vi "Dresden R2R Sputter 03.02.2018 IY24.vi"() -> ()   [LabVIEW 2009] (continued)
                                n18827 = local write "Error Message"("Shut Down Process  cancelled\nbecause  CH-VBV  not opened.\nPlease check CH-VBV2 connections." ("Error Message")) -> ()
                                n18828 = local write "Semi"(TRUE ("Semi")) -> ()
                                }
                                }
                                n18829 = local read "Ch2_Ch_vbv_di"() -> (w25328:bool)
                                n18830 = case shown="False" w25328 {
                                tunnel: [FALSE TRUE] -> w25330
                                frame #0 {
                                n18831 = local write "Ch2_Ch_vbv_do"(TRUE ("Ch1_Ch_cc_on_off_di")) -> ()
                                n18832 = Wait Until Next ms Multiple(millisecond multiple=u32 500) -> ()  [unwired: 1 out]
                                }
                                frame #1 {
                                }
                                }
                                n18833 = local read "Semi"() -> (w25331:bool)
                                n18834 = Or(x=w25330, y=w25331) -> (x .or. y?=w25329:bool)
                                }
                                }
                                frame #1 {
                                }
                                }
                                }
                                frame #1 {
                                n18835 = local read "Semi"() -> (w25341:bool)
                                n18836 = case shown="False" w25341 {
                                frame #0 {
                                n18837 = local write "Ch2_Sd13"(TRUE ("Ch1_Sd12")) -> ()
                                n18838 = Wait (ms)(milliseconds to wait=u32 1000) -> ()  [unwired: 1 out]
                                }
                                frame #1 {
                                }
                                }
                                }
                                }
                                }
                                frame #1 {
                                }
                                }
                                }
                                }
                              }
                              frame #13 {
                                # "TRNS GV-BP2 OPEN"
                                n18839 = local read "Yes 2"() -> (w25344:bool)
                                n18840 = case shown="True" w25344 {
                                frame #0 {
                                }
                                frame #1 {
                                n18841 = local read "Semi"() -> (w25345:bool)
                                n18842 = case shown="False" w25345 {
                                frame #0 {
                                n18843 = stacked-sequence {
                                frame #0 {
                                n18844 = local read "Semi"() -> (w25346:bool)
                                n18845 = case shown="False" w25346 {
                                frame #0 {
                                n18846 = while {
                                i -> [w25354]
                                stop <- w25351 stop-if-true
                                n18847 = Greater?(x=w25354, y=800) -> (0:w25353:bool)
                                n18848 = case shown="True" w25353 {
                                frame #0 {
                                }
                                frame #1 {
                                n18849 = local write "Error Message"("Shut Down process was cancelled.\nPlease check Trns GV-BP2\n connections." ("Error Message")) -> ()
                                n18850 = local write "Semi"(TRUE ("Semi")) -> ()
                                }
                                }
                                n18851 = local read "Ch2_pressure"() -> (w25349:dbl)
                                n18852 = Greater Or Equal?(x=w25349, y=700.0) -> (x >= y?=w25347:bool)
                                n18853 = case shown="False" w25347 {
                                tunnel: [FALSE w25358] -> w25350
                                frame #0 {
                                n18854 = Wait Until Next ms Multiple(millisecond multiple=u32 500) -> ()  [unwired: 1 out]
                                }
                                frame #1 {
                                n18855 = local read "Ch2_trns_gv_bp2_di"() -> (w25359:bool)
                                n18856 = case shown="False" w25359 {
                                tunnel: [FALSE TRUE] -> w25358
                                frame #0 {
                                n18857 = local write "Ch2_trns_gv_bp2_do"(TRUE ("Ch1_Trns_gv_bp2_do")) -> ()
                                n18858 = Wait Until Next ms Multiple(millisecond multiple=u32 500) -> ()  [unwired: 1 out]
                                }
                                frame #1 {
                                }
                                }
                                }
                                }
                                n18859 = local read "Semi"() -> (w25352:bool)
                                n18860 = Or(x=w25350, y=w25352) -> (x .or. y?=w25351:bool)
                                }
                                }
                                frame #1 {
                                }
                                }
                                }
                                frame #1 {
                                n18861 = local read "Semi"() -> (w25366:bool)
                                n18862 = case shown="False" w25366 {
                                frame #0 {
                                n18863 = local write "Ch2_Sd14"(TRUE ("Ch2_Sd0 14")) -> ()
                                n18864 = Wait (ms)(milliseconds to wait=u32 1000) -> ()  [unwired: 1 out]
                                }
                                frame #1 {
                                }
                                }
                                }
                                frame #2 {
                                n18865 = local read "Semi"() -> (w25369:bool)
                                n18866 = case shown="False" w25369 {
                                frame #0 {
                                n18867 = Wait (ms)(milliseconds to wait=u32 2000) -> ()  [unwired: 1 out]
                                }
                                frame #1 {
                                }
                                }
                                }
                                }
                                }
                                frame #1 {
                                }
                                }
                                }
                                }
                              }
                              frame #14 {
                                # "TRNS GV-BP OPEN"
                                n18868 = local read "Yes 2"() -> (w25371:bool)
                                n18869 = case shown="True" w25371 {
                                frame #0 {
                                }
                                frame #1 {
                                n18870 = local read "Semi"() -> (w25372:bool)
                                n18871 = case shown="False" w25372 {
                                frame #0 {
                                n18872 = stacked-sequence {
                                frame #0 {
                                n18873 = local read "Semi"() -> (w25373:bool)
                                n18874 = case shown="False" w25373 {
                                frame #0 {
                                n18875 = while {
                                i -> [w25381]
                                stop <- w25378 stop-if-true
                                n18876 = Greater?(x=w25381, y=800) -> (0:w25380:bool)
                                n18877 = case shown="True" w25380 {
                                frame #0 {
                                }
                                frame #1 {
                                n18878 = local write "Error Message"("Shut Down process was cancelled.\nPlease check Trns GV-BP\n connections." ("Error Message")) -> ()
                                n18879 = local write "Semi"(TRUE ("Semi")) -> ()
                                }
                                }
                                n18880 = local read "Ch2_pressure"() -> (w25376:dbl)
                                n18881 = Greater Or Equal?(x=w25376, y=700.0) -> (x >= y?=w25374:bool)
                                n18882 = case shown="True" w25374 {
                                tunnel: [FALSE w25385] -> w25377
                                frame #0 {
                                n18883 = Wait Until Next ms Multiple(millisecond multiple=u32 500) -> ()  [unwired: 1 out]
                                }
                                frame #1 {
                                n18884 = local read "Ch2_trns_gv_bp_di"() -> (w25386:bool)
                                n18885 = case shown="False" w25386 {
                                tunnel: [FALSE TRUE] -> w25385
                                frame #0 {
                                n18886 = local write "Ch2_trns_gv_bp_do"(TRUE ("Ch1_Trns_gv_bp2_do")) -> ()
                                n18887 = Wait Until Next ms Multiple(millisecond multiple=u32 500) -> ()  [unwired: 1 out]
                                }
                                frame #1 {
                                }
                                }
                                }
                                }
                                n18888 = local read "Semi"() -> (w25379:bool)
                                n18889 = Or(x=w25377, y=w25379) -> (x .or. y?=w25378:bool)
                                }
                                }
                                frame #1 {
                                }
                                }
                                }
                                frame #1 {
                                n18890 = local read "Semi"() -> (w25393:bool)
                                n18891 = case shown="False" w25393 {
                                frame #0 {
                                n18892 = local write "Ch2_Sd17"(TRUE ("Ch2_Sd0 15")) -> ()
                                n18893 = Wait (ms)(milliseconds to wait=u32 1000) -> ()  [unwired: 1 out]
                                }
                                frame #1 {
                                }
                                }
                                }
                                frame #2 {
                                n18894 = local read "Semi"() -> (w25396:bool)
                                n18895 = case shown="False" w25396 {
                                frame #0 {
                                n18896 = Wait (ms)(milliseconds to wait=u32 2000) -> ()  [unwired: 1 out]
                                }
                                frame #1 {
                                }
                                }
                                }
                                }
                                }
                                frame #1 {
                                }
                                }
                                }
                                }
                              }
                              frame #15 {
                                # "CH-ATM OPEN &  CHECK"
                                n18897 = local read "Yes 2"() -> (w25398:bool)
                                n18898 = case shown="True" w25398 {
                                frame #0 {
                                }
                                frame #1 {
                                n18899 = local read "Semi"() -> (w25399:bool)
                                n18900 = case shown="False" w25399 {
                                frame #0 {
                                n18901 = stacked-sequence {
                                frame #0 {
                                n18902 = local read "Semi"() -> (w25400:bool)
                                n18903 = case shown="False" w25400 {
                                frame #0 {
                                n18904 = while {
                                i -> [w25406]
                                stop <- w25403 stop-if-true
                                n18905 = Greater?(x=w25406, y=1700) -> (0:w25405:bool)
                                n18906 = case shown="True" w25405 {
                                frame #0 {
                                }
                                frame #1 {
                                n18907 = local write "Error Message"("Shut Down process was cancelled.\nPlease check Chamber \nvacuum connections." ("Error Message")) -> ()
                                n18908 = local write "Semi"(TRUE ("Semi")) -> ()
                                }
                                }
                                n18909 = local read "Ch2_Ch_atm_di"() -> (w25402:bool)
                                n18910 = case shown="False" w25402 {
                                tunnel: [FALSE TRUE] -> w25401
                                frame #0 {
                                n18911 = Wait Until Next ms Multiple(millisecond multiple=u32 500) -> ()  [unwired: 1 out]
                                }
                                frame #1 {
                                }
                                }
                                n18912 = local read "Semi"() -> (w25404:bool)
                                n18913 = Or(x=w25401, y=w25404) -> (x .or. y?=w25403:bool)
                                }
                                }
                                frame #1 {
                                }
                                }
                                }
                                frame #1 {
                                n18914 = local read "Semi"() -> (w25413:bool)
                                n18915 = case shown="False" w25413 {
                                frame #0 {
                                n18916 = local write "Ch2_Sd18"(TRUE ("Ch1_Sd10")) -> ()
                                n18917 = Wait (ms)(milliseconds to wait=u32 1000) -> ()  [unwired: 1 out]
                                }
                                frame #1 {
                                }
                                }
                                }
                                frame #2 {
                                n18918 = local read "Semi"() -> (w25416:bool)
                                n18919 = case shown="False" w25416 {
                                frame #0 {
                                n18920 = Wait (ms)(milliseconds to wait=u32 2000) -> ()  [unwired: 1 out]
                                }
                                frame #1 {
                                }
                                }
                                }
                                }
                                }
                                frame #1 {
                                }
                                }
                                }
                                }
                              }
                              frame #16 {
                                # "TRNS GV-BP2 CLOSE &  CHECK"
                                n18921 = local read "Semi"() -> (w25418:bool)
                                n18922 = case shown="False" w25418 {
                                frame #0 {
                                n18923 = stacked-sequence {
                                frame #0 {
                                n18924 = local read "Semi"() -> (w25419:bool)
                                n18925 = case shown="False" w25419 {
                                frame #0 {
                                n18926 = while {
                                i -> [w25425]
                                stop <- w25421 stop-if-true
                                n18927 = Greater?(x=w25425, y=50) -> (0:w25424:bool)
                                n18928 = case shown="True" w25424 {
                                frame #0 {
                                }
                                frame #1 {
                                n18929 = local write "Error Message"("Shut Down Process  cancelled\nbecause  Trns-GV-BP2  not closed.\nPlease check Trns-GV-BP2  connections." ("Error Message")) -> ()
                                n18930 = local write "Semi"(TRUE ("Semi")) -> ()
                                }
                                }
                                n18931 = local read "Ch2_trns_gv_bp2_di"() -> (w25420:bool)
                                n18932 = case shown="True" w25420 {
                                tunnel: [TRUE FALSE] -> w25422
                                frame #0 {
                                }
                                frame #1 {
                                n18933 = Wait Until Next ms Multiple(millisecond multiple=u32 500) -> ()  [unwired: 1 out]
                                n18934 = local write "Ch2_trns_gv_bp2_do"(FALSE ("Ch1_Ch_cc_on_off_di")) -> ()
                                }
                                }
                                n18935 = local read "Semi"() -> (w25423:bool)
                                n18936 = Or(x=w25422, y=w25423) -> (x .or. y?=w25421:bool)
                                }
                                }
                                frame #1 {
                                }
                                }
                                }
                                frame #1 {
                                n18937 = local read "Semi"() -> (w25433:bool)
                                n18938 = case shown="False" w25433 {
                                frame #0 {
                                n18939 = local write "Ch2_Sd15"(TRUE ("Ch1_Sd10 3")) -> ()
                                n18940 = Wait (ms)(milliseconds to wait=u32 1000) -> ()  [unwired: 1 out]
                                }
                                frame #1 {
                                }
                                }
                                }
                                }
                                }
                                frame #1 {
                                }
                                }
                              }
                              frame #17 {
                                # "TRNS GV-BP CLOSE &  CHECK"
                                n18941 = local read "Semi"() -> (w25436:bool)
                                n18942 = case shown="False" w25436 {
                                frame #0 {
                                n18943 = stacked-sequence {
                                frame #0 {
                                n18944 = local read "Semi"() -> (w25437:bool)
                                n18945 = case shown="False" w25437 {
                                frame #0 {
                                n18946 = while {
                                i -> [w25443]
                                stop <- w25439 stop-if-true
                                n18947 = Greater?(x=w25443, y=50) -> (0:w25442:bool)
                                n18948 = case shown="True" w25442 {
                                frame #0 {
                                }
                                frame #1 {
                                n18949 = local write "Error Message"("Shut Down Process  cancelled\nbecause  Trns-GV-BP  not closed.\nPlease check Trns-GV-BP  connections." ("Error Message")) -> ()
                                n18950 = local write "Semi"(TRUE ("Semi")) -> ()
                                }
                                }
                                n18951 = local read "Ch2_trns_gv_bp_di"() -> (w25438:bool)
                                n18952 = case shown="True" w25438 {
                                tunnel: [TRUE FALSE] -> w25440
                                frame #0 {
                                }
                                frame #1 {
                                n18953 = Wait Until Next ms Multiple(millisecond multiple=u32 500) -> ()  [unwired: 1 out]
                                n18954 = local write "Ch2_trns_gv_bp_do"(FALSE ("Ch1_Ch_cc_on_off_di")) -> ()
                                }
                                }
                                n18955 = local read "Semi"() -> (w25441:bool)
                                n18956 = Or(x=w25440, y=w25441) -> (x .or. y?=w25439:bool)
                                }
                                }
                                frame #1 {
                                }
                                }
                                }
                                frame #1 {
                                n18957 = local read "Semi"() -> (w25451:bool)
                                n18958 = case shown="False" w25451 {
                                frame #0 {
                                n18959 = local write "Ch2_Sd16"(TRUE ("Ch1_Sd10 3")) -> ()
                                n18960 = Wait (ms)(milliseconds to wait=u32 1000) -> ()  [unwired: 1 out]
                                }
                                frame #1 {
                                }
                                }
                                }
                                }
                                }
                                frame #1 {
                                }
                                }
                              }
                              frame #18 {
                                # "CH-VBV CLOSE &  CHECK"
                                n18961 = local read "Yes 2"() -> (w25454:bool)
                                n18962 = case shown="True" w25454 {
                                frame #0 {
                                }
                                frame #1 {
                                n18963 = local read "Semi"() -> (w25455:bool)
                                n18964 = case shown="False" w25455 {
                                frame #0 {
                                n18965 = stacked-sequence {
                                frame #0 {
                                n18966 = local read "Semi"() -> (w25456:bool)
                                n18967 = case shown="False" w25456 {
                                frame #0 {
                                n18968 = while {
                                i -> [w25466]
                                stop <- w25462 stop-if-true
                                n18969 = Greater?(x=w25466, y=50) -> (0:w25465:bool)
                                n18970 = case shown="True" w25465 {
                                frame #0 {
                                }
                                frame #1 {
                                n18971 = local write "Error Message"("Shut Down Process  cancelled\nbecause  CH-VBV  not closed.\nPlease check CH-VB2 connections." ("Error Message")) -> ()
                                n18972 = local write "Semi"(TRUE ("Semi")) -> ()
                                }
                                }
                                n18973 = local read "Tp2_speed_gui"() -> (w25460:i32)
                                n18974 = local read "Yes 2"() -> (w25459:bool)
                                n18975 = Greater Or Equal?(x=w25460, y=u64 100) -> (x >= y?=w25458:bool)
                                n18976 = And(x=w25459, y=w25458) -> (x .and. y?=w25457:bool)
                                n18977 = case shown="True" w25457 {
                                tunnel: [TRUE w25469] -> w25463
                                frame #0 {
                                }
                                frame #1 {
                                n18978 = local read "Ch2_Ch_vbv_di"() -> (w25470:bool)
                                n18979 = case shown="True" w25470 {
                                tunnel: [TRUE FALSE] -> w25469
                                frame #0 {
                                }
                                frame #1 {
                                n18980 = Wait Until Next ms Multiple(millisecond multiple=u32 500) -> ()  [unwired: 1 out]
                                n18981 = local write "Ch2_Ch_vbv_do"(FALSE ("Ch1_Ch_cc_on_off_di")) -> ()
                                }
                                }
                                }
                                }
                                n18982 = local read "Semi"() -> (w25464:bool)
                                n18983 = Or(x=w25463, y=w25464) -> (x .or. y?=w25462:bool)
                                }
                                }
                                frame #1 {
                                }
                                }
                                }
                                frame #1 {
                                n18984 = local read "Semi"() -> (w25477:bool)
                                n18985 = case shown="False" w25477 {
                                frame #0 {
                                n18986 = local write "Ch2_Sd19"(TRUE ("Ch1_Sd10 2")) -> ()
                                n18987 = Wait (ms)(milliseconds to wait=u32 1000) -> ()  [unwired: 1 out]
                                }
                                frame #1 {
                                }
                                }
                                }
                                frame #2 {
                                n18988 = local read "Semi"() -> (w25480:bool)
                                n18989 = case shown="False" w25480 {
                                frame #0 {
                                n18990 = Wait (ms)(milliseconds to wait=u32 3000) -> ()  [unwired: 1 out]
                                }
                                frame #1 {
                                }
                                }
                                }
                                }
                                }
                                frame #1 {
                                }
                                }
                                }
                                }
                              }
                              frame #19 {
                                # "CLOSE PC-BV"
                                n18991 = local read "Yes 2"() -> (w25482:bool)
                                n18992 = case shown="True" w25482 {
                                frame #0 {
                                }
                                frame #1 {
                                n18993 = local read "Semi"() -> (w25483:bool)
                                n18994 = case shown="False" w25483 {
                                frame #0 {
                                n18995 = stacked-sequence {
                                frame #0 {
                                n18996 = local read "Semi"() -> (w25484:bool)
                                n18997 = case shown="False" w25484 {
                                frame #0 {
                                n18998 = stacked-sequence {
                                frame #0 {
                                n18999 = local read "Semi"() -> (w25485:bool)
                                n19000 = case shown="False" w25485 {
                                frame #0 {
                                n19001 = local write "Pc_bv2_auto_close"(TRUE ("Tp1_auto_start")) -> ()
                                }
                                frame #1 {
                                }
                                }
                                }
                                frame #1 {
                                n19002 = local read "Semi"() -> (w25487:bool)
                                n19003 = case shown="False" w25487 {
                                frame #0 {
                                n19004 = Wait (ms)(milliseconds to wait=u32 1000) -> ()  [unwired: 1 out]
                                }
                                frame #1 {
                                }
                                }
                                }
                                frame #2 {
                                n19005 = local read "Semi"() -> (w25489:bool)
                                n19006 = case shown="False" w25489 {
                                frame #0 {
                                n19007 = while {
                                i -> [w25495]
                                stop <- w25491 stop-if-true
                                n19008 = local read "Pc_bv_closed_ch2"() -> (w25493:bool)
                                n19009 = Greater?(x=w25495, y=120) -> (0:w25494:bool)
                                n19010 = local read "Semi"() -> (w25492:bool)
                                n19011 = Compound Arithmetic op=OR(w25492, w25493, w25494) -> (w25491:bool)
                                n19012 = Wait (ms)(milliseconds to wait=u32 500) -> ()  [unwired: 1 out]
                                }
                                }
                                frame #1 {
                                }
                                }
                                }
                                frame #3 {
                                n19013 = local read "Semi"() -> (w25497:bool)
                                n19014 = case shown="False" w25497 {
                                frame #0 {
                                n19015 = local read "Pc_bv_closed_ch2"() -> (w25498:bool)
                                n19016 = case shown="False" w25498 {
                                frame #0 {
                                n19017 = local write "Pc_bv2_auto_close"(TRUE ("Pc_bv1_auto_open")) -> ()
                                }
                                frame #1 {
                                }
                                }
                                }
                                frame #1 {
                                }
                                }
                                }
                                frame #4 {
                                n19018 = local read "Semi"() -> (w25500:bool)
                                n19019 = case shown="False" w25500 {
                                frame #0 {
                                n19020 = local read "Pc_bv_closed_ch2"() -> (w25501:bool)
                                n19021 = case shown="False" w25501 {
                                frame #0 {
                                n19022 = Wait (ms)(milliseconds to wait=u32 1000) -> ()  [unwired: 1 out]
                                }
                                frame #1 {
                                }
                                }
                                }
                                frame #1 {
                                }
                                }
                                }
                                frame #5 {
                                n19023 = local read "Semi"() -> (w25503:bool)
                                n19024 = case shown="False" w25503 {
                                frame #0 {
                                n19025 = while {
                                i -> [w25509]
                                stop <- w25505 stop-if-true
                                n19026 = local read "Pc_bv_closed_ch2"() -> (w25507:bool)
                                n19027 = Greater?(x=w25509, y=120) -> (0:w25508:bool)
                                n19028 = local read "Semi"() -> (w25506:bool)
                                n19029 = Compound Arithmetic op=OR(w25506, w25507, w25508) -> (w25505:bool)
                                n19030 = Wait (ms)(milliseconds to wait=u32 500) -> ()  [unwired: 1 out]
                                }
                                }
                                frame #1 {
                                }
                                }
                                }
                                frame #6 {
                                n19031 = local read "Semi"() -> (w25511:bool)
                                n19032 = case shown="False" w25511 {
                                frame #0 {
                                n19033 = local read "Pc_bv_closed_ch2"() -> (w25512:bool)
                                n19034 = case shown="False" w25512 {
                                frame #0 {
                                n19035 = local write "Error Message"("Shut Down process  cancelled\nbecause  PC-BV not closed.\nPlease check PC-BV2 connections." ("Error Message")) -> ()
                                n19036 = Wait (ms)(milliseconds to wait=u32 1000) -> ()  [unwired: 1 out]
                                }
                                frame #1 {
                                }
                                }
                                }
                                frame #1 {
                                }
                                }
                                }
                                }
                                }
                                frame #1 {
                                }
                                }
                                }
                                frame #1 {
                                n19037 = local read "Semi"() -> (w25515:bool)
                                n19038 = case shown="False" w25515 {
                                frame #0 {
                                n19039 = Wait (ms)(milliseconds to wait=u32 1000) -> ()  [unwired: 1 out]
                                n19040 = local write "Ch2_Sd20"(TRUE ("Ch1_Sd14")) -> ()
                                }
                                frame #1 {
                                }
                                }
                                }
                                }
                                }
                                frame #1 {
                                }
                                }
                                }
                                }
                              }
                              frame #20 {
                                # "CH-VBV CLOSE &  CHECK"
                                n19041 = local read "Semi"() -> (w25518:bool)
                                n19042 = case shown="False" w25518 {
                                frame #0 {
                                n19043 = stacked-sequence {
                                frame #0 {
                                n19044 = local read "Semi"() -> (w25519:bool)
                                n19045 = case shown="False" w25519 {
                                frame #0 {
                                n19046 = while {
                                i -> [w25525]
                                stop <- w25521 stop-if-true
                                n19047 = Greater?(x=w25525, y=50) -> (0:w25524:bool)
                                n19048 = case shown="True" w25524 {
                                frame #0 {
                                }
                                frame #1 {
                                n19049 = local write "Error Message"("Shut Down Process  cancelled\nbecause  CH-VBV  not closed.\nPlease check CH-VBV2 connections." ("Error Message")) -> ()
                                n19050 = local write "Semi"(TRUE ("Semi")) -> ()
                                }
                                }
                                n19051 = local read "Ch2_Ch_vbv_di"() -> (w25520:bool)
                                n19052 = case shown="True" w25520 {
                                tunnel: [TRUE FALSE] -> w25522
                                frame #0 {
                                }
                                frame #1 {
                                n19053 = Wait Until Next ms Multiple(millisecond multiple=u32 500) -> ()  [unwired: 1 out]
                                n19054 = local write "Ch2_Ch_vbv_do"(FALSE ("Ch1_Ch_cc_on_off_di")) -> ()
                                }
                                }
                                n19055 = local read "Semi"() -> (w25523:bool)
                                n19056 = Or(x=w25522, y=w25523) -> (x .or. y?=w25521:bool)
                                }
                                }
                                frame #1 {
                                }
                                }
                                }
                                frame #1 {
                                n19057 = local read "Semi"() -> (w25533:bool)
                                n19058 = case shown="False" w25533 {
                                frame #0 {
                                n19059 = local write "Ch2_Sd21"(TRUE ("Ch1_Sd10 3")) -> ()
                                n19060 = Wait (ms)(milliseconds to wait=u32 1000) -> ()  [unwired: 1 out]
                                }
                                frame #1 {
                                }
                                }
                                }
                                }
                                }
                                frame #1 {
                                }
                                }
                              }
                              frame #21 {
                                # "FINISH SHUTDOWN"
                                n19061 = local read "Semi"() -> (w25536:bool)
                                n19062 = case shown="False" w25536 {
                                frame #0 {
                                n19063 = stacked-sequence {
                                frame #0 {
                                n19064 = local read "Semi"() -> (w25537:bool)
                                n19065 = case shown="False" w25537 {
                                frame #0 {
                                w25538 = TRUE ("Visible")
                                n19066 = property on="final_mes_tab" class="TabCtl (strict)"("Visible"=w25538) -> ()  [unwired: 2 in, 2 out]
                                n19067 = local write "Cnt_Do_Buzzer"(w25538) -> ()
                                n19068 = local write "system_status"(" CH2 Shut Down Process was completed." ("system_status")) -> ()
                                n19069 = Wait (ms)(milliseconds to wait=u32 3000) -> ()  [unwired: 1 out]
                                }
                                frame #1 {
                                }
                                }
                                }
                                frame #1 {
                                n19070 = local read "Semi"() -> (w25541:bool)
                                n19071 = case shown="False" w25541 {
                                frame #0 {
                                w25542 = FALSE ("Visible")
                                n19072 = property on="final_mes_tab" class="TabCtl (strict)"("Visible"=w25542) -> ()  [unwired: 2 in, 2 out]
                                n19073 = local write "Shutdown_ch2"(w25542) -> ()
                                n19074 = local write "Cnt_Do_Buzzer"(w25542) -> ()
                                n19075 = local write "system_status"("" ("system_status")) -> ()
                                n19076 = Wait (ms)(milliseconds to wait=u32 3000) -> ()  [unwired: 1 out]
                                }
                                frame #1 {
                                }
                                }
                                }
                                frame #2 {
                                n19077 = local read "Semi"() -> (w25545:bool)
                                n19078 = case shown="False" w25545 {
                                frame #0 {
                                n19079 = stacked-sequence {
                                frame #0 {
                                n19080 = local write "Pps_code_entry"("PF233=" ("Pps_code_entry")) -> ()
                                }
                                frame #1 {
                                n19081 = Wait (ms)(milliseconds to wait=u32 500) -> ()  [unwired: 1 out]
                                }
                                frame #2 {
                                n19082 = local write "Ppsok"(TRUE ("Ppsok")) -> ()
                                }
                                frame #3 {
                                n19083 = Wait (ms)(milliseconds to wait=u32 500) -> ()  [unwired: 1 out]
                                }
                                }
                                }
                                frame #1 {
                                }
                                }
                                }
                                frame #3 {
                                n19084 = local read "Semi"() -> (w25550:bool)
                                n19085 = case shown="False" w25550 {
                                frame #0 {
                                n19086 = stacked-sequence {
                                frame #0 {
                                n19087 = local write "Pps_code_entry"("PF234=" ("Pps_code_entry")) -> ()
                                }
                                frame #1 {
                                n19088 = Wait (ms)(milliseconds to wait=u32 500) -> ()  [unwired: 1 out]
                                }
                                frame #2 {
                                n19089 = local write "Ppsok"(TRUE ("Ppsok")) -> ()
                                }
                                frame #3 {
                                n19090 = Wait (ms)(milliseconds to wait=u32 500) -> ()  [unwired: 1 out]
                                }
                                }
                                }
                                frame #1 {
                                }
                                }
                                }
                                frame #4 {
                                n19091 = local read "Semi"() -> (w25555:bool)
                                n19092 = case shown="False" w25555 {
                                frame #0 {
                                n19093 = local write "Ch2_Sd22"(TRUE ("Ch1_Sd15")) -> ()
                                n19094 = Wait (ms)(milliseconds to wait=u32 500) -> ()  [unwired: 1 out]
                                }
                                frame #1 {
                                }
                                }
                                }
                                }
                                }
                                frame #1 {
                                }
                                }
                              }
                            }
                          }
                        }
                      }
                    }
                  }
                  frame #1 {
                  }
                }
              }
            }
          }
          frame #1 {
          }
        }
      }
    }
    n19095 = case shown="True" "Start_up_ch3" {
      frame #0 {
      }
      frame #1 {
        # "START UP OF CH3 PROCEDURE"
        n19096 = stacked-sequence {
          frame #0 {
            # "ROUTINE CHECK"
            n19097 = local read "Semi"() -> (w23827:bool)
            n19098 = case shown="False" w23827 {
              frame #0 {
                n19099 = stacked-sequence {
                  frame #0 {
                    n19100 = local write "Clean_Pumping_ch3"(TRUE) -> ()
                    n19101 = local write "final_process_messages"("Start up process was completed." ("final_process_messages")) -> ()
                    n19102 = property on="Pressure_time_graph_ch3" class="WFChart (strict)"("History Data"=dbl[] []) -> ()  [unwired: 2 in, 2 out]
                    n19103 = local write "system_status"("Start up process continues." ("system_status")) -> ()
                    n19104 = Wait (ms)(milliseconds to wait=u32 1000) -> ()  [unwired: 1 out]
                  }
                  frame #1 {
                    n19105 = local read "Semi"() -> (w23833:bool)
                    n19106 = case shown="False" w23833 {
                      frame #0 {
                        n19107 = stacked-sequence {
                          frame #0 {
                            n19108 = local read "Semi"() -> (w23834:bool)
                            n19109 = case shown="False" w23834 {
                              frame #0 {
                                n19110 = while {
                                i -> [w23841]